vi "Dresden R2R Sputter 03.02.2018 IY24.vi"() -> ()   [LabVIEW 2009] (continued)
                  }
                }
              }
            }
            n286 = case shown="True" "Ch1_Cst_fix_up" {
              frame #0 {
              }
              frame #1 {
                n287 = stacked-sequence {
                  frame #0 {
                    n288 = local write "Ch1_Cst_fix_do"(i16? 0 ("Ch1_Trns_gv_open_do")) -> ()
                  }
                }
              }
            }
            n289 = stacked-sequence {
              frame #0 {
                n290 = case shown="True" "Ch2_Pet_cool_up" {
                  frame #0 {
                  }
                  frame #1 {
                    n291 = stacked-sequence {
                      frame #0 {
                        n292 = local write "Ch2_Pet_cool_down_do"(i16? 0 ("Ch1_Trns_gv_open_do")) -> ()
                      }
                      frame #1 {
                        n293 = local write "Ch2_Pet_cool_up_do"(T/1 ("Ch1_Trns_gv_open_do")) -> ()
                      }
                    }
                  }
                }
                n294 = case shown="True" "Ch2_Pet_cool_down" {
                  frame #0 {
                  }
                  frame #1 {
                    n295 = stacked-sequence {
                      frame #0 {
                        n296 = local write "Ch2_Pet_cool_up_do"(i16? 0 ("Ch1_Trns_gv_open_do")) -> ()
                      }
                      frame #1 {
                        n297 = local write "Ch2_Pet_cool_down_do"(T/1 ("Ch1_Trns_gv_open_do")) -> ()
                      }
                    }
                  }
                }
              }
            }
            n298 = case shown="True" "Ch2_Cst_fix_down" {
              frame #0 {
              }
              frame #1 {
                n299 = stacked-sequence {
                  frame #0 {
                    n300 = local write "Ch2_Cst_fix_do"(T/1 ("Ch1_Trns_gv_open_do")) -> ()
                  }
                }
              }
            }
            n301 = case shown="True" "Ch2_Cst_fix_up" {
              frame #0 {
              }
              frame #1 {
                n302 = stacked-sequence {
                  frame #0 {
                    n303 = local write "Ch2_Cst_fix_do"(i16? 0 ("Ch1_Trns_gv_open_do")) -> ()
                  }
                }
              }
            }
            n304 = stacked-sequence {
              frame #0 {
                n305 = case shown="True" "Ch3_Pet_cool_up" {
                  frame #0 {
                  }
                  frame #1 {
                    n306 = stacked-sequence {
                      frame #0 {
                        n307 = local write "Ch3_Pet_cool_down_do"(i16? 0 ("Ch1_Trns_gv_open_do")) -> ()
                      }
                      frame #1 {
                        n308 = local write "Ch3_Pet_cool_up_do"(T/1 ("Ch1_Trns_gv_open_do")) -> ()
                      }
                    }
                  }
                }
                n309 = case shown="True" "Ch3_Pet_cool_down" {
                  frame #0 {
                  }
                  frame #1 {
                    n310 = stacked-sequence {
                      frame #0 {
                        n311 = local write "Ch3_Pet_cool_up_do"(i16? 0 ("Ch1_Trns_gv_open_do")) -> ()
                      }
                      frame #1 {
                        n312 = local write "Ch3_Pet_cool_down_do"(T/1 ("Ch1_Trns_gv_open_do")) -> ()
                      }
                    }
                  }
                }
              }
            }
            n313 = case shown="True" "Ch3_Cst_fix_up" {
              frame #0 {
              }
              frame #1 {
                n314 = stacked-sequence {
                  frame #0 {
                    n315 = local write "Ch3_Cst_fix_do"(i16? 0 ("Ch1_Trns_gv_open_do")) -> ()
                  }
                }
              }
            }
            n316 = case shown="True" "Ch3_Cst_fix_down" {
              frame #0 {
              }
              frame #1 {
                n317 = stacked-sequence {
                  frame #0 {
                    n318 = local write "Ch3_Cst_fix_do"(T/1 ("Ch1_Trns_gv_open_do")) -> ()
                  }
                }
              }
            }
            n319 = stacked-sequence {
              frame #0 {
                n320 = case shown="True" "Ch4_Pet_cool_up" {
                  frame #0 {
                  }
                  frame #1 {
                    n321 = stacked-sequence {
                      frame #0 {
                        n322 = local write "Ch4_Pet_cool_down_do"(i16? 0 ("Ch1_Trns_gv_open_do")) -> ()
                      }
                      frame #1 {
                        n323 = local write "Ch4_Pet_cool_up_do"(T/1 ("Ch1_Trns_gv_open_do")) -> ()
                      }
                    }
                  }
                }
                n324 = case shown="True" "Ch4_Pet_cool_down" {
                  frame #0 {
                  }
                  frame #1 {
                    n325 = stacked-sequence {
                      frame #0 {
                        n326 = local write "Ch4_Pet_cool_up_do"(i16? 0 ("Ch1_Trns_gv_open_do")) -> ()
                      }
                      frame #1 {
                        n327 = local write "Ch4_Pet_cool_down_do"(T/1 ("Ch1_Trns_gv_open_do")) -> ()
                      }
                    }
                  }
                }
              }
            }
            n328 = case shown="True" "Ch4_Cst_fix_down" {
              frame #0 {
              }
              frame #1 {
                n329 = stacked-sequence {
                  frame #0 {
                    n330 = local write "Ch4_Cst_fix_do"(T/1 ("Ch1_Trns_gv_open_do")) -> ()
                  }
                }
              }
            }
            n331 = case shown="True" "Ch4_Cst_fix_up" {
              frame #0 {
              }
              frame #1 {
                n332 = stacked-sequence {
                  frame #0 {
                    n333 = local write "Ch4_Cst_fix_do"(i16? 0 ("Ch1_Trns_gv_open_do")) -> ()
                  }
                }
              }
            }
          }
        }
        n334 = stacked-sequence {
          frame #0 {
            n335 = stacked-sequence {
              frame #0 {
                n336 = Compound Arithmetic op=OR("Ch1_Trns_gv_bp2_open_gui", "Ch1_Trns_gv_bp2_open", "Ch1_Trns_gv_bp_front_open gui", "Ch1_Trns_gv_bp_top_open_gui", "Ch1_Trns_gv_bp_top_open") -> (w1462)
                n337 = Compound Arithmetic op=OR("Ch1_Trns_gv_bp2_close_gui", "Ch1_Trns_gv_bp2_close", "Ch1_Trns_gv_bp_front_close gui", "Ch1_Trns_gv_bp_top_close gui", "Ch1_Trns_gv_bp_top_close") -> (w1459)
                n338 = case shown="True" w1462 {
                  frame #0 {
                  }
                  frame #1 {
                    n339 = local read "Ch1_Trns_gv_bp2_open_safety"() -> (w1464)
                    n340 = case shown="False" w1464 {
                      frame #0 {
                        n341 = local write "Error Message"("Trns GV-BP2 can not be opened.                   \nReason : * CH1 pressure can not\n be atmospheric.       \n           *CH1 and CH2 pressure \ncan not be less than 0.9 torr." ("Error Message")) -> ()
                      }
                      frame #1 {
                        n342 = local write "Ch1_Trns_gv_bp2_do"(T/1 ("Ch3_Do_Bp_bv_L")) -> ()
                      }
                    }
                  }
                }
                n343 = case shown="True" w1459 {
                  frame #0 {
                  }
                  frame #1 {
                    n344 = local write "Ch1_Trns_gv_bp2_do"(i16? 0 ("Ch3_Do_Bp_bv_L")) -> ()
                  }
                }
              }
            }
            n345 = stacked-sequence {
              frame #0 {
                n346 = Compound Arithmetic op=OR("Ch3_Trns_gv_bp_open_gui", "Ch3_Trns_gv_bp_open", "Ch3_Trns_gv_bp_front_open gui", "Ch3_Trns_gv_bp_top_open gui", "Ch3_Trns_gv_bp_top_open") -> (w1445)
                n347 = Compound Arithmetic op=OR("Ch3_Trns_gv_bp_close_gui", "Ch3_Trns_gv_bp_close", "Ch3_Trns_gv_bp_front_close_gui", "Ch3_Trns_gv_bp_top_close_gui", "Ch3_Trns_gv_bp_top_close") -> (w1446)
                n348 = case shown="True" w1445 {
                  frame #0 {
                  }
                  frame #1 {
                    n349 = local read "Ch3_Trns_gv_bp_open_safety"() -> (w1448)
                    n350 = case shown="False" w1448 {
                      frame #0 {
                        n351 = local write "Error Message"("Trns GV-BP can not be opened.  \nReason : * CH3 pressure can not be\n atmospheric.                      \n           *CH3 and CH2 pressure can not be\n less than 0.9 torr." ("Error Message")) -> ()
                      }
                      frame #1 {
                        n352 = local write "Ch3_Trns_gv_bp_do"(T/1 ("Ch3_Do_Bp_bv_L")) -> ()
                      }
                    }
                  }
                }
                n353 = case shown="True" w1446 {
                  frame #0 {
                  }
                  frame #1 {
                    n354 = local write "Ch3_Trns_gv_bp_do"(i16? 0 ("Ch3_Do_Bp_bv_L")) -> ()
                  }
                }
              }
            }
            n355 = stacked-sequence {
              frame #0 {
                n356 = Compound Arithmetic op=OR("Ch2_Trns_gv_bp2_top_open", "Ch2_Trns_gv_bp2_open_gui", "Ch2_Trns_gv_bp2_open", "Ch2_Trns_gv_bp2_front_open_gui", "Ch2_Trns_gv_bp2_top_open") -> (w1429)
                n357 = Compound Arithmetic op=OR("Ch2_Trns_gv_bp2_close_gui", "Ch2_Trns_gv_bp2_close", "Ch2_Trns_gv_bp2_top_close", "Ch2_Trns_gv_bp2_front_close_gui", "Ch2_Trns_gv_bp2_top_close") -> (w1430)
                n358 = case shown="True" w1430 {
                  frame #0 {
                  }
                  frame #1 {
                    n359 = local write "Ch2_trns_gv_bp2_do"(i16? 0 ("Ch3_Do_Bp_bv_L")) -> ()
                  }
                }
                n360 = case shown="True" w1429 {
                  frame #0 {
                  }
                  frame #1 {
                    n361 = local read "Ch2_Trns_gv_bp2_open_safety"() -> (w1432)
                    n362 = case shown="False" w1432 {
                      frame #0 {
                        n363 = local write "Error Message"("Trns GV-BP2 can not be opened.    \nReason : * CH2 pressure can not \nbe atmospheric           \n           *CH2 and CH3 pressure can not be\n less than 0.9 torr." ("Error Message")) -> ()
                      }
                      frame #1 {
                        n364 = local write "Ch2_trns_gv_bp2_do"(T/1 ("Ch3_Do_Bp_bv_L")) -> ()
                      }
                    }
                  }
                }
              }
            }
            n365 = stacked-sequence {
              frame #0 {
                n366 = Compound Arithmetic op=OR("Ch4_Trns_gv_bp_close_gui", "Ch4_Trns_gv_bp_close", "Ch4_Trns_gv_bp_front close gui", "Ch4_Trns_gv_bp_top_close", "Ch4_Trns_gv_bp_top_close gui") -> (w1414)
                n367 = Compound Arithmetic op=OR("Ch4_Trns_gv_bp_open_gui", "Ch4_Trns_gv_bp_open", "Ch4_Trns_gv_bp_top_open", "Ch4_Trns_gv_bp_open top_gui", "Ch4_Trns_gv_bp_front_open gui") -> (w1413)
                n368 = case shown="True" w1414 {
                  frame #0 {
                  }
                  frame #1 {
                    n369 = local write "Ch4_Trns_gv_bp_do"(i16? 0 ("Ch3_Do_Bp_bv_L")) -> ()
                  }
                }
                n370 = case shown="True" w1413 {
                  frame #0 {
                  }
                  frame #1 {
                    n371 = local read "Ch4_Trns_gv_bp_close_safety"() -> (w1416)
                    n372 = case shown="False" w1416 {
                      frame #0 {
                        n373 = local write "Error Message"("Trns GV-BP can not be opened. \nReason : * CH3 pressure can not be\n atmospheric.                      \n           *CH4 and CH3 pressure can not be\n less than 0.9 torr." ("Error Message")) -> ()
                      }
                      frame #1 {
                        n374 = local write "Ch4_Trns_gv_bp_do"(T/1 ("Ch3_Do_Bp_bv_L")) -> ()
                      }
                    }
                  }
                }
              }
            }
            n375 = stacked-sequence {
              frame #0 {
                n376 = Compound Arithmetic op=OR("Ch2_Trns_gv_bp_top_open_ gui", "Ch2_Trns_gv_bp_front_open", "Ch2_Trns_gv_bp_open_gui", "Ch2_Trns_gv_bp_open", "Ch2_Trns_gv_bp_top_open") -> (w1382)
                n377 = Compound Arithmetic op=OR("Ch2_Trns_gv_bp_top_close", "Ch2_Trns_gv_bp_close_gui", "Ch2_Trns_gv_bp_front_close_gui", "Ch2_Trns_gv_bp_close_gui", "Ch2_Trns_gv_bp_close") -> (w1381)
                n378 = case shown="True" w1381 {
                  frame #0 {
                  }
                  frame #1 {
                    n379 = local write "Ch2_trns_gv_bp_do"(i16? 0 ("Ch3_Do_Bp_bv_L")) -> ()
                  }
                }
                n380 = case shown="True" w1382 {
                  frame #0 {
                  }
                  frame #1 {
                    n381 = local read "Ch2_Trns_gv_bp_open_safety"() -> (w1384)
                    n382 = case shown="False" w1384 {
                      frame #0 {
                        n383 = local write "Error Message"("Trns GV-BP can not be opened.  \nReason : * CH2 pressure can not be \natmospheric.                      \n           *CH2 and CH1 pressure can not be\n less than 0.9 torr." ("Error Message")) -> ()
                      }
                      frame #1 {
                        n384 = local write "Ch2_trns_gv_bp_do"(T/1 ("Ch3_Do_Bp_bv_L")) -> ()
                      }
                    }
                  }
                }
              }
            }
            n385 = stacked-sequence {
              frame #0 {
                n386 = Compound Arithmetic op=OR("Ch3_Trns_gv_bp2_open_gui", "Ch3_Trns_gv_bp2_open", "Ch3_Trns_gv_bp2_top_open", "Ch3_Trns_gv_bp2_top_open_gui", "Ch3_Trns_gv_bp2_front_open") -> (w1398)
                n387 = Compound Arithmetic op=OR("Ch3_Trns_gv_bp2_close_gui", "Ch3_Trns_gv_bp2_close", "Ch3_Trns_gv_bp2_top_close", "Ch3_Trns_gv_bp2_top_close_gui", "Ch3_Trns_gv_bp2_front close gui") -> (w1397)
                n388 = case shown="True" w1398 {
                  frame #0 {
                  }
                  frame #1 {
                    n389 = local read "Ch3_Trns_gv_bp2_open_safety"() -> (w1400)
                    n390 = case shown="False" w1400 {
                      frame #0 {
                        n391 = local write "Error Message"("Trns GV-BP2 can not be opened. \nReason : * CH3 pressure can not be\n atmospheric.                      \n           *CH3 and CH4 pressure can not be \nless than 0.9 torr." ("Error Message")) -> ()
                      }
                      frame #1 {
                        n392 = local write "Ch3_Trns_gv_bp2_do"(T/1 ("Ch3_Do_Bp_bv_L")) -> ()
                      }
                    }
                  }
                }
                n393 = case shown="True" w1397 {
                  frame #0 {
                  }
                  frame #1 {
                    n394 = local write "Ch3_Trns_gv_bp2_do"(i16? 0 ("Ch3_Do_Bp_bv_L")) -> ()
                  }
                }
              }
            }
          }
        }
        n395 = stacked-sequence {
          frame #0 {
            n396 = stacked-sequence {
              frame #0 {
                n397 = case shown="True" "Ch1_Srv_pist_back" {
                  frame #0 {
                  }
                  frame #1 {
                    n398 = stacked-sequence {
                      frame #0 {
                        n399 = local write "Ch1_SRV1_PIST For_do"(i16? 0 ("Ch1_Trns_gv_open_do")) -> ()
                      }
                      frame #1 {
                        n400 = local write "Ch1_SRV1_PIST_Back_do"(T/1 ("Ch1_Trns_gv_open_do")) -> ()
                      }
                    }
                  }
                }
                n401 = case shown="True" "Ch1_Srv_pist_for" {
                  frame #0 {
                  }
                  frame #1 {
                    n402 = stacked-sequence {
                      frame #0 {
                        n403 = local write "Ch1_SRV1_PIST_Back_do"(i16? 0 ("Ch1_Trns_gv_open_do")) -> ()
                      }
                      frame #1 {
                        n404 = local write "Ch1_SRV1_PIST For_do"(T/1 ("Ch1_Trns_gv_open_do")) -> ()
                      }
                    }
                  }
                }
              }
            }
            n405 = stacked-sequence {
              frame #0 {
                n406 = case shown="True" "Ch2_Srv_pist_back" {
                  frame #0 {
                  }
                  frame #1 {
                    n407 = stacked-sequence {
                      frame #0 {
                        n408 = local write "Ch1_SRV1_PIST For_do"(i16? 0 ("Ch1_Trns_gv_open_do")) -> ()
                      }
                      frame #1 {
                        n409 = local write "Ch2_SRV1_PIST_Back_do"(T/1 ("Ch1_Trns_gv_open_do")) -> ()
                      }
                    }
                  }
                }
                n410 = case shown="True" "Ch2_Srv_pist_for" {
                  frame #0 {
                  }
                  frame #1 {
                    n411 = stacked-sequence {
                      frame #0 {
                        n412 = local write "Ch2_SRV1_PIST_Back_do"(i16? 0 ("Ch1_Trns_gv_open_do")) -> ()
                      }
                      frame #1 {
                        n413 = local write "Ch2_SRV1_PIST For_do"(T/1 ("Ch1_Trns_gv_open_do")) -> ()
                      }
                    }
                  }
                }
              }
            }
            n414 = stacked-sequence {
              frame #0 {
                n415 = case shown="True" "Ch3_Srv_pist_for" {
                  frame #0 {
                  }
                  frame #1 {
                    n416 = stacked-sequence {
                      frame #0 {
                        n417 = local write "Ch3_SRV1_PIST_Back_do"(i16? 0 ("Ch1_Trns_gv_open_do")) -> ()
                      }
                      frame #1 {
                        n418 = local write "Ch3_SRV1_PIST For_do"(T/1 ("Ch1_Trns_gv_open_do")) -> ()
                      }
                    }
                  }
                }
                n419 = case shown="True" "Ch3_Srv_pist_back" {
                  frame #0 {
                  }
                  frame #1 {
                    n420 = stacked-sequence {
                      frame #0 {
                        n421 = local write "Ch3_SRV1_PIST For_do"(i16? 0 ("Ch1_Trns_gv_open_do")) -> ()
                      }
                      frame #1 {
                        n422 = local write "Ch3_SRV1_PIST_Back_do"(T/1 ("Ch1_Trns_gv_open_do")) -> ()
                      }
                    }
                  }
                }
              }
            }
            n423 = stacked-sequence {
              frame #0 {
                n424 = case shown="True" "Ch4_Srv_pist_for" {
                  frame #0 {
                  }
                  frame #1 {
                    n425 = stacked-sequence {
                      frame #0 {
                        n426 = local write "Ch4_SRV1_PIST_Back_do"(i16? 0 ("Ch1_Trns_gv_open_do")) -> ()
                      }
                      frame #1 {
                        n427 = local write "Ch4_SRV1_PIST For_do"(T/1 ("Ch1_Trns_gv_open_do")) -> ()
                      }
                    }
                  }
                }
                n428 = case shown="True" "Ch4_Srv_pist_back" {
                  frame #0 {
                  }
                  frame #1 {
                    n429 = stacked-sequence {
                      frame #0 {
                        n430 = local write "Ch4_SRV1_PIST For_do"(i16? 0 ("Ch1_Trns_gv_open_do")) -> ()
                      }
                      frame #1 {
                        n431 = local write "Ch4_SRV1_PIST_Back_do"(T/1 ("Ch1_Trns_gv_open_do")) -> ()
                      }
                    }
                  }
                }
              }
            }
          }
        }
        n432 = stacked-sequence {
          frame #0 {
            n433 = stacked-sequence {
              frame #0 {
                n434 = Compound Arithmetic op=OR("Gv_top_ch2_1_open gui", "Gv_open ch1_2_gui", "Gv_open ch1_2_tab", "Gv_front_ch2_1_open_gui", "Gv_front_ch1_2_open gui", "Gv_top_ch1_2_open", "Gv_top_ch1_2_open gui", "Gv_top_ch2_1_open", "Gv_open ch1_2_tab 2") -> (w1366)
                n435 = Compound Arithmetic op=OR("Gv_top_ch2_1_close gui", "Gv_front_ch1_2_close gui", "Gv_top_ch1_2_close", "Gv_top_ch1_2_close gui", "Gv_close_ch1_2_gui", "Gv_close_ch1_2tab", "Gv_front_ch2_1_close_gui", "Gv_top_ch2_1_close", "Gv_close_ch1_2tab 2") -> (w1365)
                n436 = case shown="True" w1366 {
                  frame #0 {
                  }
                  frame #1 {
                    n437 = stacked-sequence {
                      frame #0 {
                        n438 = local write "Ch1_Trns_gv_close_do"(i16? 0 ("Ch1_Trns_gv_open_do")) -> ()
                      }
                      frame #1 {
                        n439 = local write "Ch1_Trns_gv_open_do"(T/1 ("Ch1_Trns_gv_open_do")) -> ()
                      }
                    }
                  }
                }
                n440 = case shown="True" w1365 {
                  frame #0 {
                  }
                  frame #1 {
                    n441 = stacked-sequence {
                      frame #0 {
                        n442 = local write "Ch1_Trns_gv_open_do"(i16? 0 ("Ch1_Trns_gv_open_do")) -> ()
                      }
                      frame #1 {
                        n443 = local write "Ch1_Trns_gv_close_do"(T/1 ("Ch1_Trns_gv_close_do")) -> ()
                      }
                    }
                  }
                }
              }
            }
            n444 = stacked-sequence {
              frame #0 {
                n445 = Compound Arithmetic op=OR("Gv_top_ch2_3_open_gui", "Gv_top_ch3_2_open", "Gv_top_open_3_2 gui", "Gv_front_ch3_2_open_gui", "Gv_front_ch2_3_open gui", "Gv_open ch2_3_gui", "Gv_open ch2_3tab", "Gv_front_ch3_2_open", "Gv_open ch2_3tab 2") -> (w1338)
                n446 = Compound Arithmetic op=OR("Gv_front_ch3_2_close", "Gv_top_ch2_3_close gui", "Gv_top_ch3_2_close", "Gv_front_ch3_2_close_gui", "Gv_top_ch3_2_close_gui", "Gv_front_ch2_3_close gui", "Gv_close_ch2_3_gui", "Gv_close_ch2_3tab", "Gv_close_ch2_3tab 2") -> (w1333)
                n447 = case shown="True" w1338 {
                  frame #0 {
                  }
                  frame #1 {
                    n448 = stacked-sequence {
                      frame #0 {
                        n449 = local write "Ch2_Trns_gv_close_do"(i16? 0 ("Ch2_Trns_gv_close_do")) -> ()
                      }
                      frame #1 {
                        n450 = local write "Ch2_Trns_gv_open_do"(T/1 ("Ch2_Trns_gv_open_do")) -> ()
                      }
                    }
                  }
                }
                n451 = case shown="True" w1333 {
                  frame #0 {
                  }
                  frame #1 {
                    n452 = stacked-sequence {
                      frame #0 {
                        n453 = local write "Ch2_Trns_gv_open_do"(i16? 0 ("Ch2_Trns_gv_open_do")) -> ()
                      }
                      frame #1 {
                        n454 = local write "Ch2_Trns_gv_close_do"(T/1 ("Ch2_Trns_gv_close_do")) -> ()
                      }
                    }
                  }
                }
              }
            }
            n455 = stacked-sequence {
              frame #0 {
                n456 = Compound Arithmetic op=OR("Gv_open ch3_4tab 2", "Gv_open ch3_4gui", "Gv_open ch3_4tab", "Gv_front_ch3_4_open", "Gv_front_ch3_4_open", "Gv_front_ch3_4_open_gui", "Gv_top_ch3_4_open  gui", "Gv_top_ch3_4_open_gui", "Gv_front_ch3_4_open_gui") -> (w1318)
                n457 = Compound Arithmetic op=OR("Gv_front_ch3_4_close", "Gv_front_ch3_4_close gui", "Gv_top_ch3_4_close gui", "Gv_top_ch3_4_close_gui", "Gv_close_ch3_4gui", "Gv_close_ch3_4tab", "Gv_front_ch3_4_close", "Gv_front_ch3_4_close_gui", "Gv_close_ch3_4tab 2") -> (w1317)
                n458 = case shown="True" w1317 {
                  frame #0 {
                  }
                  frame #1 {
                    n459 = stacked-sequence {
                      frame #0 {
                        n460 = local write "Ch3_Trns_gv_open_do"(i16? 0 ("Ch2_Trns_gv_open_do")) -> ()
                      }
                      frame #1 {
                        n461 = local write "Ch3_Trns_gv_close_do"(T/1 ("Ch2_Trns_gv_close_do")) -> ()
                      }
                    }
                  }
                }
                n462 = case shown="True" w1318 {
                  frame #0 {
                  }
                  frame #1 {
                    n463 = stacked-sequence {
                      frame #0 {
                        n464 = local write "Ch3_Trns_gv_close_do"(i16? 0 ("Ch2_Trns_gv_close_do")) -> ()
                      }
                      frame #1 {
                        n465 = local write "Ch3_Trns_gv_open_do"(T/1 ("Ch2_Trns_gv_open_do")) -> ()
                      }
                    }
                  }
                }
              }
            }
          }
        }
        n466 = Wait Until Next ms Multiple(millisecond multiple=i32? 300) -> ()  [unwired: 1 out]
        n467 = stacked-sequence {
          frame #0 {
            n468 = Or(x="Ch1_Pl_vbv_open_gui", y="Ch1_Pl_vbv_open") -> (x .or. y?=w1724)
            n469 = Or(x="Ch1_Pl_vbv_close_gui", y="Ch1_Pl_vbv_close") -> (x .or. y?=w1723)
            n470 = case shown="True" w1724 {
              frame #0 {
              }
              frame #1 {
                n471 = local read "Ch1_Pl_vbv_open_safety"() -> (w1747)
                n472 = case shown="True" w1747 {
                  frame #0 {
                    n473 = local write "Error Message"("PL-VBV can not be opened.\nReason :  *MPcan not be stopped.\n*TP-BV can be open.       " ("Error Message")) -> ()
                  }
                  frame #1 {
                    n474 = stacked-sequence {
                      frame #0 {
                        n475 = local write "Ch1_Pl_atm_do"(i16? 0 ("Ch1_Ch_vbv_do")) -> ()
                      }
                      frame #1 {
                        n476 = Wait (ms)(milliseconds to wait=i32? 500) -> ()  [unwired: 1 out]
                      }
                      frame #2 {
                        n477 = local write "Ch1_Pl_vbv_do"(T/1 ("Ch1_Ch_vbv_do")) -> ()
                      }
                      frame #3 {
                        n478 = Wait (ms)(milliseconds to wait=i32? 500) -> ()  [unwired: 1 out]
                      }
                    }
                  }
                }
              }
            }
            n479 = case shown="True" w1723 {
              frame #0 {
              }
              frame #1 {
                n480 = local write "Ch1_Pl_vbv_do"(i16? 0 ("Ch1_Pl_vbv_do")) -> ()
              }
            }
            n481 = Or(x="Ch2_Pl_vbv_stop_gui", y="Ch2_Pl_vbv_stop") -> (x .or. y?=w1722)
            n482 = Or(x="Ch2_Pl_vbv_start_gui", y="Ch2_Pl_vbv_start") -> (x .or. y?=w1721)
            n483 = case shown="True" w1721 {
              frame #0 {
              }
              frame #1 {
                n484 = local read "Ch2_Pl_vbv_open_safety"() -> (w1740)
                n485 = case shown="True" w1740 {
                  frame #0 {
                    n486 = local write "Error Message"("PL-VBV can not be opened.\nReason :  *MPcan not be stopped.\n*TP-BV can be open.       " ("Error Message")) -> ()
                  }
                  frame #1 {
                    n487 = stacked-sequence {
                      frame #0 {
                        n488 = local write "Ch2_Pl_atm_do"(i16? 0 ("Ch1_Ch_vbv_do")) -> ()
                      }
                      frame #1 {
                        n489 = Wait (ms)(milliseconds to wait=i32? 500) -> ()  [unwired: 1 out]
                      }
                      frame #2 {
                        n490 = local write "Ch2_Pl_vbv_do"(T/1 ("Ch1_Ch_vbv_do")) -> ()
                      }
                      frame #3 {
                        n491 = Wait (ms)(milliseconds to wait=i32? 500) -> ()  [unwired: 1 out]
                      }
                    }
                  }
                }
              }
            }
            n492 = case shown="True" w1722 {
              frame #0 {
              }
              frame #1 {
                n493 = local write "Ch2_Pl_vbv_do"(i16? 0 ("Ch1_Pl_vbv_do")) -> ()
              }
            }
            n494 = Or(x="Ch3_Pl_vbv_start_gui", y="Ch3_Pl_vbv_start_tab") -> (x .or. y?=w1710)
            n495 = Or(x="Ch3_Pl_vbv_stop_gui", y="Ch3_Pl_vbv_stop_tab") -> (x .or. y?=w1707)
            n496 = case shown="True" w1710 {
              frame #0 {
              }
              frame #1 {
                n497 = local read "Ch3_Pl_vbv_open_safety"() -> (w1733)
                n498 = case shown="True" w1733 {
                  frame #0 {
                    n499 = local write "Error Message"("PL-VBV can not be opened.\nReason :  *MPcan not be stopped.\n*TP-BV can be open.       " ("Error Message")) -> ()
                  }
                  frame #1 {
                    n500 = stacked-sequence {
                      frame #0 {
                        n501 = local write "Ch3_Pl_atm_do"(i16? 0 ("Ch1_Ch_vbv_do")) -> ()
                      }
                      frame #1 {
                        n502 = Wait (ms)(milliseconds to wait=i32? 500) -> ()  [unwired: 1 out]
                      }
                      frame #2 {
                        n503 = local write "Ch3_Pl_vbv_do"(T/1 ("Ch1_Ch_vbv_do")) -> ()
                      }
                      frame #3 {
                        n504 = Wait (ms)(milliseconds to wait=i32? 500) -> ()  [unwired: 1 out]
                      }
                    }
                  }
                }
              }
            }
            n505 = case shown="True" w1707 {
              frame #0 {
              }
              frame #1 {
                n506 = local write "Ch3_Pl_vbv_do"(i16? 0 ("Ch1_Pl_vbv_do")) -> ()
              }
            }
            n507 = Or(x="Ch4_Pl_vbv_start_gui", y="Ch4_Pl_vbv_start_tab") -> (x .or. y?=w1705)
            n508 = Or(x="Ch4_Pl_vbv_stop_gui", y="Ch4_Pl_vbv_stop_tab") -> (x .or. y?=w1703)
            n509 = case shown="True" w1705 {
              frame #0 {
              }
              frame #1 {
                n510 = local read "Ch4_Pl_vbv_open_safety"() -> (w1726)
                n511 = case shown="True" w1726 {
                  frame #0 {
                    n512 = local write "Error Message"("PL-VBV can not be opened.\nReason :  *MPcan not be stopped.\n*TP-BV can be open.       " ("Error Message")) -> ()
                  }
                  frame #1 {
                    n513 = stacked-sequence {
                      frame #0 {
                        n514 = local write "Ch4_Pl_atm_do"(i16? 0 ("Ch1_Ch_vbv_do")) -> ()
                      }
                      frame #1 {
                        n515 = Wait (ms)(milliseconds to wait=i32? 500) -> ()  [unwired: 1 out]
                      }
                      frame #2 {
                        n516 = local write "Ch4_Pl_vbv_do"(T/1 ("Ch1_Ch_vbv_do")) -> ()
                      }
                      frame #3 {
                        n517 = Wait (ms)(milliseconds to wait=i32? 500) -> ()  [unwired: 1 out]
                      }
                    }
                  }
                }
              }
            }
            n518 = case shown="True" w1703 {
              frame #0 {
              }
              frame #1 {
                n519 = local write "Ch4_Pl_vbv_do"(i16? 0 ("Ch1_Pl_vbv_do")) -> ()
              }
            }
          }
        }
        n520 = stacked-sequence {
          frame #0 {
            n521 = Compound Arithmetic op=OR("Ch1_Bg_bv_close_gui", "Ch1_Bg_bv_close", "Ch1_bg_bv_top_close", "Ch1_bg_bv_top_close gui") -> (w1659)
            n522 = Compound Arithmetic op=OR("Ch1_Bg_bv_open_gui", "Ch1_Bg_bv_open", "Ch1_bg_bv_top_open gui", "Ch1_bg_bv_top_open") -> (w1664)
            n523 = case shown="False" w1664 {
              frame #0 {
              }
              frame #1 {
                n524 = local read "Ch1_Bg_bv_open_safety"() -> (w1698)
                n525 = case shown="True" w1698 {
                  frame #0 {
                    n526 = local write "Error Message"("BG-BV can not be opened.\nReason :  *CH pressure can be higher than 1E-1" ("Error Message")) -> ()
                  }
                  frame #1 {
                    n527 = local write "Ch1_Bg_bv_do"(T/1 ("Ch1_Bg_bv_do")) -> ()
                  }
                }
              }
            }
            n528 = case shown="True" w1659 {
              frame #0 {
              }
              frame #1 {
                n529 = local read "Ch1_Bg_bv_close_safety"() -> (w1695)
                n530 = case shown="True" w1695 {
                  frame #0 {
                    n531 = local write "Error Message"("BG-BV can not be closed.\nReason :  *PC-BV can control  \n  position or pressure." ("Error Message")) -> ()
                  }
                  frame #1 {
                    n532 = local write "Ch1_Bg_bv_do"(i16? 0 ("Ch1_Bg_bv_do")) -> ()
                  }
                }
              }
            }
            n533 = Compound Arithmetic op=OR("Ch2_Bg_bv_close_gui", "Ch2_Bg_bv_close", "Ch2_bg_bv_top_close", "Ch2_bg_bv_L_top_close") -> (w1653)
            n534 = Compound Arithmetic op=OR("Ch2_Bg_bv_open_gui", "Ch2_Bg_bv_open", "Ch2_bg_bv_top_open", "Ch2_bg_bv_top_open") -> (w1656)
            n535 = case shown="False" w1656 {
              frame #0 {
              }
              frame #1 {
                n536 = local read "Ch2_Bg_bv_open_safety"() -> (w1692)
                n537 = case shown="False" w1692 {
                  frame #0 {
                    n538 = local write "Error Message"("BG-BV can not be opened.\nReason :  *CH pressure can be higher \nthan 1E-1" ("Error Message")) -> ()
                  }
                  frame #1 {
                    n539 = local write "Ch2_Bg_bv_do"(T/1 ("Ch1_Bg_bv_do")) -> ()
                  }
                }
              }
            }
            n540 = case shown="True" w1653 {
              frame #0 {
              }
              frame #1 {
                n541 = local read "Ch2_Bg_bv_close_safety"() -> (w1689)
                n542 = case shown="False" w1689 {
                  frame #0 {
                    n543 = local write "Error Message"("BG-BV can not be closed.\nReason :  *PC-BV can control  \n  position or pressure." ("Error Message")) -> ()
                  }
                  frame #1 {
                    n544 = local write "Ch2_Bg_bv_do"(i16? 0 ("Ch1_Bg_bv_do")) -> ()
                  }
                }
              }
            }
            n545 = Compound Arithmetic op=OR("Ch3_Bg_bv_open_gui", "Ch3_Bg_bv_open", "Ch3_bg_bv_top_open gui", "Ch3_bg_bv_top_open") -> (w1665)
            n546 = Compound Arithmetic op=OR("Ch3_Bg_bv_close_gui", "Bg_bv_close_ch3", "Ch3_bg_bv_top_close_gui", "Ch3_bg_bv_top_close") -> (w1668)
            n547 = case shown="True" w1668 {
              frame #0 {
              }
              frame #1 {
                n548 = local read "Ch3_Bg_bv_close_safety"() -> (w1683)
                n549 = case shown="True" w1683 {
                  frame #0 {
                    n550 = local write "Error Message"("BG-BV can not be closed.\nReason :  *PC-BV can control  \n  position or pressure." ("Error Message")) -> ()
                  }
                  frame #1 {
                    n551 = local write "Ch3_Bg_bv_do"(i16? 0 ("Ch1_Bg_bv_do")) -> ()
                  }
                }
              }
            }
            n552 = case shown="True" w1665 {
              frame #0 {
              }
              frame #1 {
                n553 = local read "Ch3_Bg_bv_start_safety"() -> (w1686)
                n554 = case shown="False" w1686 {
                  frame #0 {
                    n555 = local write "Error Message"("BG-BV can not be opened.\nReason :  *CH pressure can be higher \nthan 1E-1" ("Error Message")) -> ()
                  }
                  frame #1 {
                    n556 = local write "Ch3_Bg_bv_do"(T/1 ("Ch1_Bg_bv_do")) -> ()
                  }
                }
              }
            }
            n557 = Compound Arithmetic op=OR("Ch4_Bg_bv_open_gui", "Ch4_Bg_bv_open", "Ch4_Bg_bv_top_open gui", "Ch4_Bg_bv_top_open") -> (w1674)
            n558 = Compound Arithmetic op=OR("Ch4_Bg_bv_close_gui", "Ch4_Bg_bv_close", "Ch4_bg_bv_top_close gui", "Ch4_bg_bv_top_close") -> (w1671)
            n559 = case shown="True" w1674 {
              frame #0 {
              }
              frame #1 {
                n560 = local read "Ch4_Bg_bv_open_safety"() -> (w1680)
                n561 = case shown="True" w1680 {
                  frame #0 {
                    n562 = local write "Error Message"("BG-BV can not be opened.\nReason :  *CH pressure can be higher \nthan 1E-1" ("Error Message")) -> ()
                  }
                  frame #1 {
                    n563 = local write "Ch4_Bg_bv_do"(T/1 ("Ch1_Bg_bv_do")) -> ()
                  }
                }
              }
            }
            n564 = case shown="True" w1671 {
              frame #0 {
              }
              frame #1 {
                n565 = local read "Ch4_Bg_bv_close_safety"() -> (w1677)
                n566 = case shown="True" w1677 {
                  frame #0 {
                    n567 = local write "Error Message"("BG-BV can not be closed.\nReason :  *PC-BV can control  \n  position or pressure." ("Error Message")) -> ()
                  }
                  frame #1 {
                    n568 = local write "Ch4_Bg_bv_do"(i16? 0 ("Ch1_Bg_bv_do")) -> ()
                  }
                }
              }
            }
          }
        }
        n569 = stacked-sequence {
          frame #0 {
            n570 = Or(x="Ch1_Tp_bv_open_gui", y="Ch1_Tp_bv_open_tab") -> (x .or. y?=w1612)
            n571 = Or(x="Ch1_Tp_bv_close_gui", y="Ch1_Tp_bv_close_tab") -> (x .or. y?=w1611)
            n572 = case shown="True" w1612 {
              frame #0 {
              }
              frame #1 {
                n573 = local read "Ch1_Tp_bv_open_safety"() -> (w1634)
                n574 = case shown="True" w1634 {
                  frame #0 {
                    n575 = local write "Error Message"("TP-BV can not be opened.\nReason : *TP can not be stopped." ("Error Message")) -> ()
                  }
                  frame #1 {
                    n576 = local write "Ch1_Tp_bv_do"(T/1 ("Ch1_Tp_bv_do")) -> ()
                  }
                }
              }
            }
            n577 = case shown="True" w1611 {
              frame #0 {
              }
              frame #1 {
                n578 = local read "Ch1_Tp_bv_close_safety"() -> (w1631)
                n579 = case shown="True" w1631 {
                  frame #0 {
                    n580 = local write "Error Message"("TP-BV can not be closed.\nReason : *Difference chamber pressure and\n pipeline pressure are not suitable.\n  " ("Error Message")) -> ()
                  }
                  frame #1 {
                    n581 = local write "Ch1_Tp_bv_do"(i16? 0 ("Ch1_Tp_bv_do")) -> ()
                  }
                }
              }
            }
            n582 = Or(x="Ch2_Tp_bv_close_gui", y="Ch2_Tp_bv close_tab") -> (x .or. y?=w1610)
            n583 = Or(x="Ch2_Tp_bv_open_gui", y="Ch2_Tp_bv_open_tab") -> (x .or. y?=w1609)
            n584 = case shown="False" w1609 {
              frame #0 {
              }
              frame #1 {
                n585 = local read "Ch2_Tp_bv_open_safety"() -> (w1628)
                n586 = case shown="False" w1628 {
                  frame #0 {
                    n587 = local write "Error Message"("TP-BV can not be opened.\nReason : *TP can not be stopped." ("Error Message")) -> ()
                  }
                  frame #1 {
                    n588 = local write "Ch2_Tp_bv_do"(T/1 ("Ch1_Tp_bv_do")) -> ()
                  }
                }
              }
            }
            n589 = case shown="True" w1610 {
              frame #0 {
              }
              frame #1 {
                n590 = local read "Ch2_Tp_bv_close_safety"() -> (w1625)
                n591 = case shown="False" w1625 {
                  frame #0 {
                    n592 = local write "Error Message"("TP-BV can not be closed.\nReason : *Difference chamber pressure and\n pipeline pressure are not suitable.\n  " ("Error Message")) -> ()
                  }
                  frame #1 {
                    n593 = local write "Ch2_Tp_bv_do"(i16? 0 ("Ch1_Tp_bv_do")) -> ()
                  }
                }
              }
            }
            n594 = Or(x="Ch3_Tp_bv_close_gui", y="Ch3_Tp_bv_close") -> (x .or. y?=w1595)
            n595 = Or(x="Ch3_Tp_bv_open_gui", y="Ch3_Tp_bv_open") -> (x .or. y?=w1598)
            n596 = case shown="True" w1598 {
              frame #0 {
              }
              frame #1 {
                n597 = local read "Ch3_Tp_bv_open_safety"() -> (w1622)
                n598 = case shown="True" w1622 {
                  frame #0 {
                    n599 = local write "Error Message"("TP-BV can not be opened.\nReason : *TP can not be stopped." ("Error Message")) -> ()
                  }
                  frame #1 {
                    n600 = local write "Ch3_Tp_bv_do"(T/1 ("Ch1_Tp_bv_do")) -> ()
                  }
                }
              }
            }
            n601 = case shown="True" w1595 {
              frame #0 {
              }
              frame #1 {
                n602 = local read "Ch3_Tp_bv_close_safety"() -> (w1619)
                n603 = case shown="True" w1619 {
                  frame #0 {
                    n604 = local write "Error Message"("TP-BV can not be closed.\nReason : *Difference chamber pressure and\n pipeline pressure are not suitable.\n  " ("Error Message")) -> ()
                  }
                  frame #1 {
                    n605 = local write "Ch3_Tp_bv_do"(i16? 0 ("Ch1_Tp_bv_do")) -> ()
                  }
                }
              }
            }
            n606 = Or(x="Ch4_Tp_bv_close_gui", y="Ch4_Tp_bv_close") -> (x .or. y?=w1589)
            n607 = Or(x="Ch4_Tp_bv_open_gui", y="Ch4_Tp_bv_open") -> (x .or. y?=w1592)
            n608 = case shown="True" w1592 {
              frame #0 {
              }
              frame #1 {
                n609 = local read "Ch4_Tp_bv_open_safety"() -> (w1616)
                n610 = case shown="True" w1616 {
                  frame #0 {
                    n611 = local write "Error Message"("TP-BV can not be opened.\nReason : *TP can not be stopped." ("Error Message")) -> ()
                  }
                  frame #1 {
                    n612 = local write "Ch4_Tp_bv_do"(T/1 ("Ch1_Tp_bv_do")) -> ()
                  }
                }
              }
            }
            n613 = case shown="True" w1589 {
              frame #0 {
              }
              frame #1 {
                n614 = local read "Ch4_Tp_bv_close_safety"() -> (w1613)
                n615 = case shown="True" w1613 {
                  frame #0 {
                    n616 = local write "Error Message"("TP-BV can not be closed.\nReason : *Difference chamber pressure and\n pipeline pressure are not suitable.\n  " ("Error Message")) -> ()
                  }
                  frame #1 {
                    n617 = local write "Ch4_Tp_bv_do"(i16? 0 ("Ch1_Tp_bv_do")) -> ()
                  }
                }
              }
            }
          }
        }
        n618 = stacked-sequence {
          frame #0 {
            n619 = disable-structure shown="Disabled" {
              frame #0 {
                n620 = stacked-sequence {
                  frame #0 {
                    n621 = Or(x="Bp_bv_open_ch3_L_gui", y="Bp_bv_open_ch3_L") -> (x .or. y?=w1484)
                    n622 = Or(x="Bp_bv_close_ch3_L_gui", y="Bp_bv_close_ch3_L") -> (x .or. y?=w1483)
                    n623 = case shown="True" w1484 {
                      frame #0 {
                      }
                      frame #1 {